vi "Main.vi"() -> ()   [LabVIEW 2020]
uses:
  System.Windows.Forms
  Global_Variable/Global.vi
  Global_Variable/A131258.vi
  Database/Global1.vi
  <userlib>/_MGI/Menu Building/MenuTypes/MenuStrip/MGI_MenuStrip.lvclass
  <userlib>/_MGI/Menu Building/MenuItemStatusChange/MGI_MenuItemStatusChange.lvclass
  Libraries/S7/S7.lvlib
panel:
  out "左空载扭矩":dbl format="%#.3f Nm"
  out "右加载扭矩":dbl format="%#.3f Nm"
  out "上序状态":string
  out "右工位传感器码":string
  in  "表格控件":string[][](table)
  in  "Andon":enum32{"未选择", "缺料报警", "质量报警", "故障报警"}(radio)
  out "PLC":bool
  in  "菜单":refnum<k24>(container)
  out "试验计时":u16
  out "工位传感器码":string
  out "生产数量":i32
  out "合格数量":i32
  out "userStatus":string caption="用户状态"
  out "userName":string caption="用户名"
  out "connectionMode":string caption="联机类型"
  out "产品型号":string
  in  "更换产品":refnum<vi>
  out "提示信息":string
  out "错误":bool
  out "时间字符串":string
  out "日期字符串":string
  out "自动":bool
  # "芯轴分总成磨合台"
  # "实验项目"
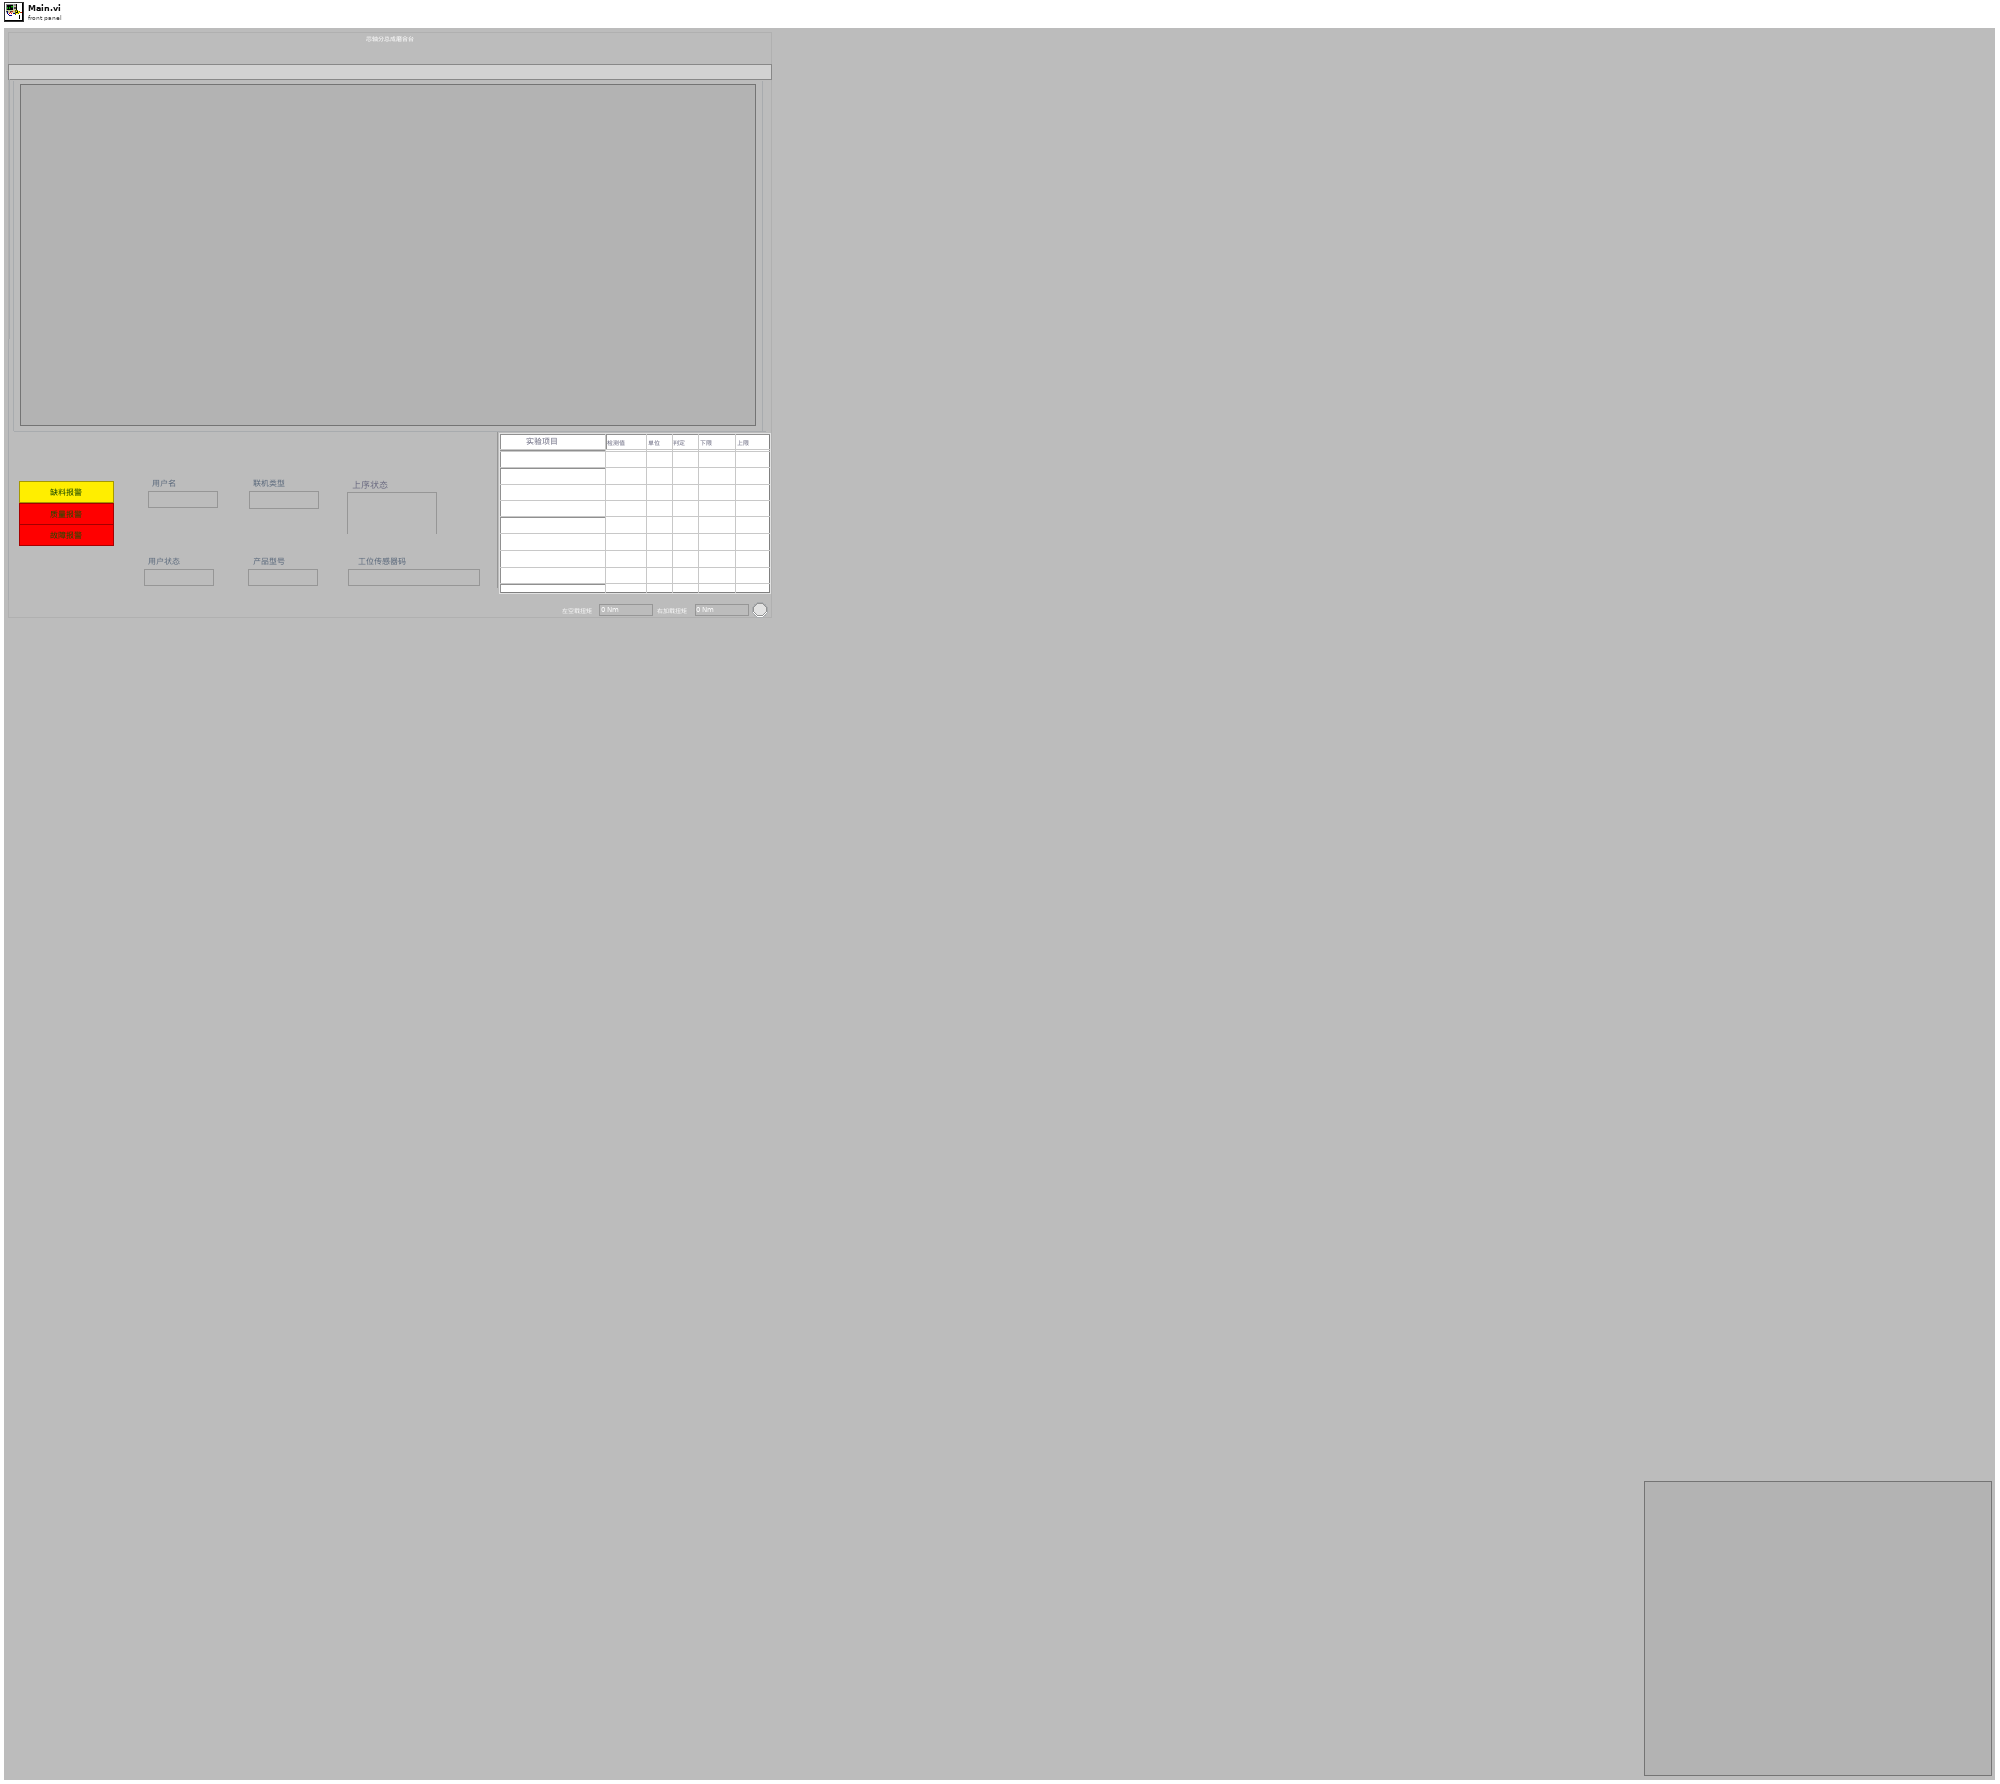
[diagram p1: front panel]
types:
  T1 = typedef "S7.lvlib/Broadcast Events--cluster.ctl" = cluster{"Module Did Init":refnum<user-event>, "Status Updated":refnum<user-event>, "Error Reported":refnum<user-event>, "Module Did Stop":refnum<user-event>, "Update Module Execution Status":refnum<user-event>}
  T2 = enum32{"Invalid", "Standard", "Closed", "Hidden", "Minimized", "Maximized"}
  T3 = cluster{"设备名称":string, "操作人员":string, "设备状态":enum16{"设备离线", "设备正常", "设备缺料", "设备故障", "质量报警"}, "附加信息":string}
  T4 = enum32{"invalid app kind", "Development System", "Run Time System", "Student Edition", "Embedded LabVIEW", "Evaluation", "Custom"}
  T5 = cluster{"左平均扭矩":cluster{"正转":dbl, "反转":dbl}, "左矩波动":cluster{"正转":dbl, "反转":dbl}, "左空载":cluster{"正转":dbl, "反转":dbl}, "右平均扭矩":cluster{"正转":dbl, "反转":dbl}, "右扭矩波动":cluster{"正转":dbl, "反转":dbl}, "右空载":cluster{"正转":dbl, "反转":dbl}, "扭矩对称":cluster{"左":dbl, "右":dbl}, "左零点漂移":cluster{"正":dbl, "反":dbl}, "右零点漂移":cluster{"正":dbl, "反":dbl}}
  T6 = cluster{"用户编号":string, "用户名":string, "用户密码(密文)":string, "用户权限":string}
  T7 = cluster{"Core":cluster{"Current VI Reference":refnum<vi>, "Close Panel on Exit?":bool}, "Your Boolean data":bool, "Your string data":string}
  T8 = cluster{"Current VI Reference":refnum<vi>, "Close Panel on Exit?":bool}
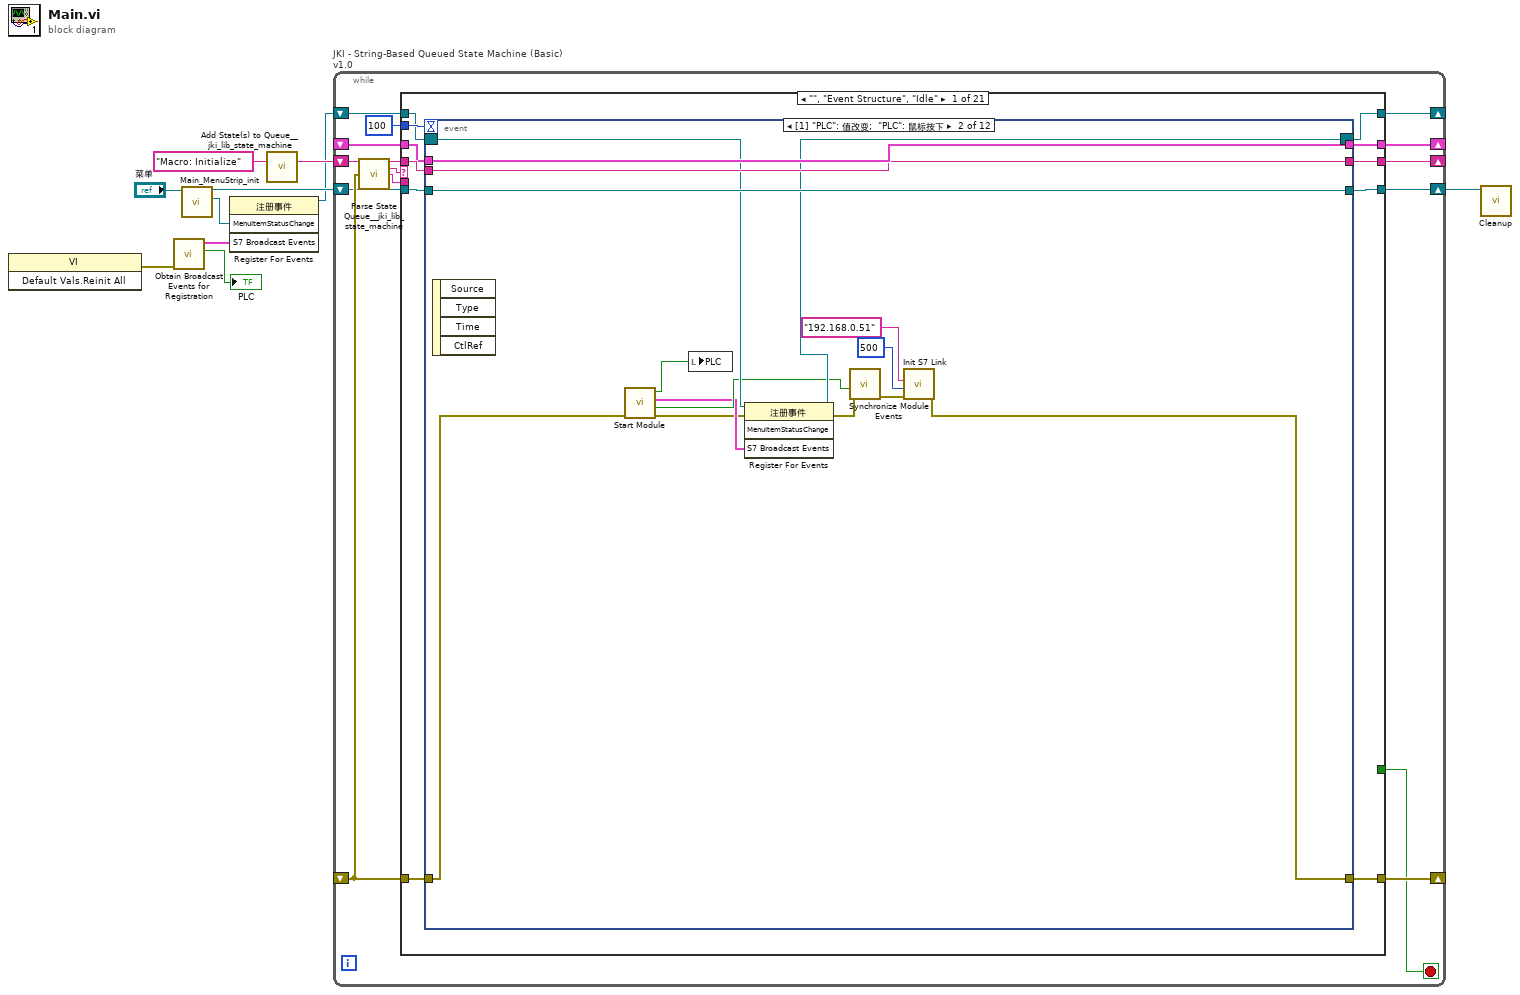
[diagram p0: block diagram]
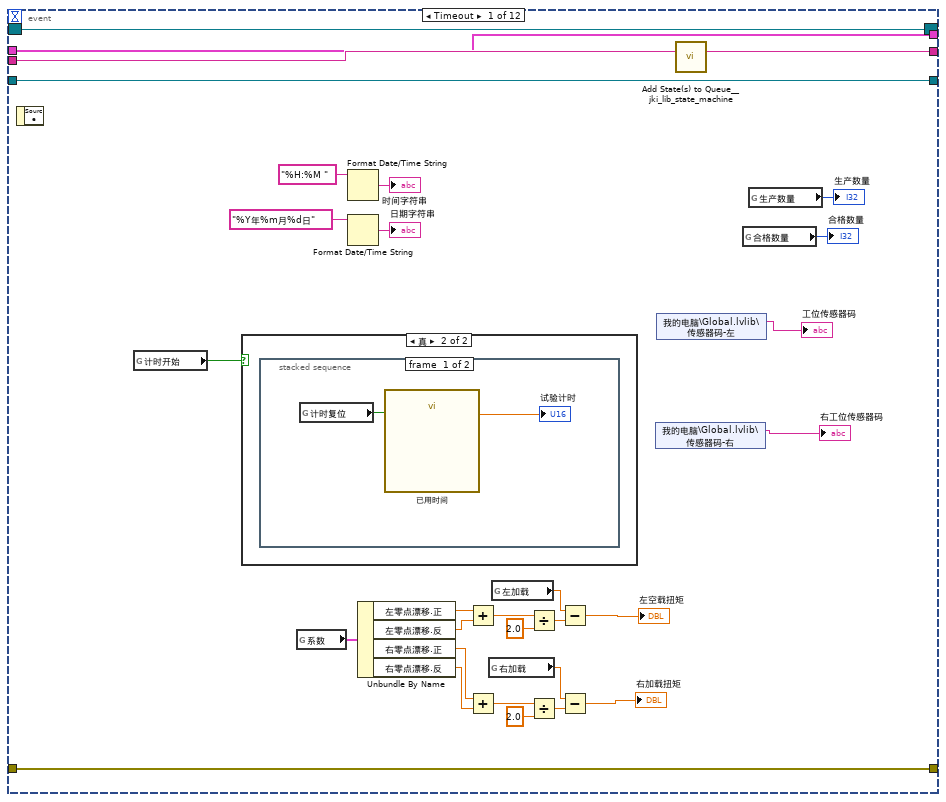
[diagram p2: hidden frame]
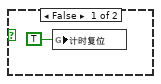
[diagram p3: hidden frame]
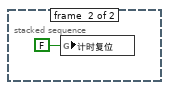
[diagram p4: hidden frame]
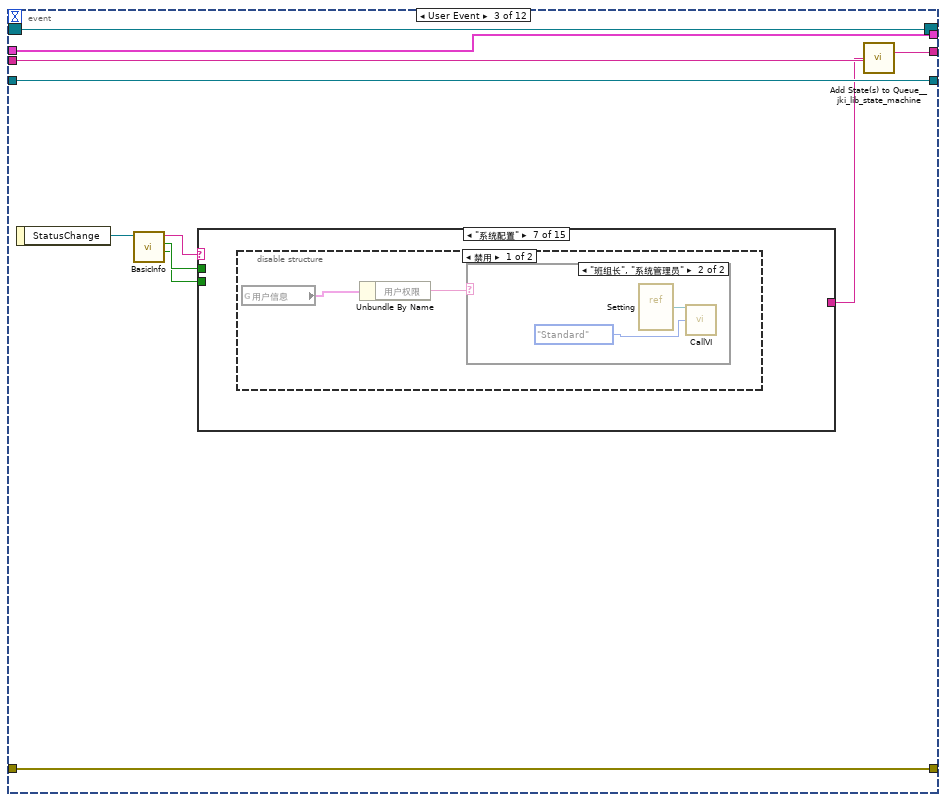
[diagram p5: hidden frame]
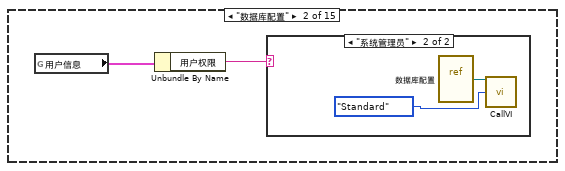
[diagram p7: hidden frame]
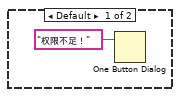
[diagram p8: hidden frame]
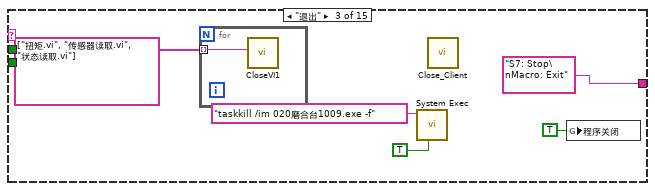
[diagram p9: hidden frame]
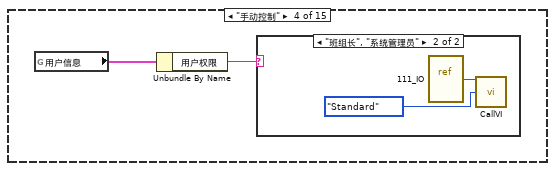
[diagram p10: hidden frame]
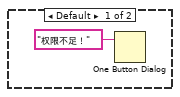
[diagram p11: hidden frame]
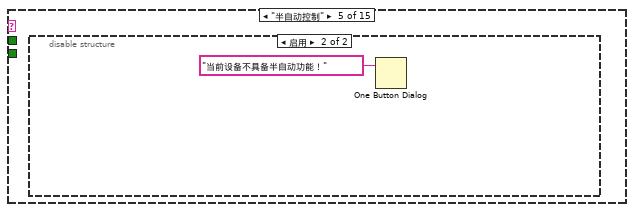
[diagram p12: hidden frame]
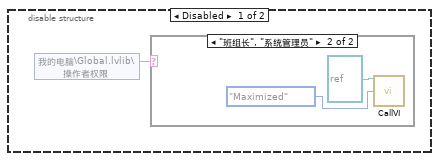
[diagram p13: hidden frame]
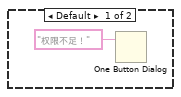
[diagram p14: hidden frame]
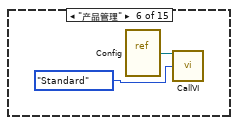
[diagram p15: hidden frame]
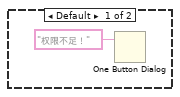
[diagram p16: hidden frame]
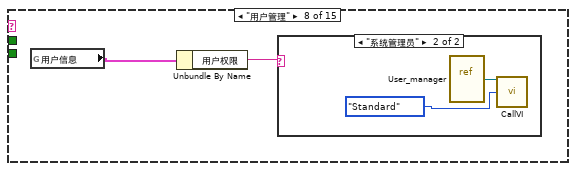
[diagram p18: hidden frame]
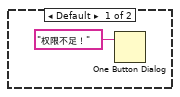
[diagram p19: hidden frame]
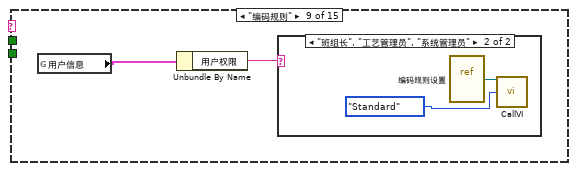
[diagram p20: hidden frame]
diagram:
  n1 = invoke class="VI" method="Default Vals.Reinit All"() -> (error out=w3:errorcluster)  [unwired: 3 in, 2 out]
  n2 = call "Obtain Broadcast Events for Registration.vi"("error in (no error)"=w3) -> ("Already running?"=→"PLC":bool, "S7 Broadcast Events"=w5:T1)  [unwired: 8 in, 1 out]
  n3 = call "Main_MenuStrip_init.vi"("MenuStrip"="菜单") -> ("MenuItemStatusChange"=w2:refnum<user-event>, "Menu out"=w7:refnum<class "MGI_MenuStrip.lvclass">)  [unwired: 9 in]
  n4 = register-events(w2, w5) -> (reference out=w1:refnum<event-registration>)  [unwired: 2 in, 1 out]
  n5 = call <vilib>:"Add State(s) to Queue__jki_lib_state_machine.vi"("State(s) in (\"\")"="Macro: Initialize") -> ("States Out"=w10:string)  [unwired: 14 in]
  n6 = while "JKI - String-Based Queued State Machine (Basic) v1.0" {
    shift-right: [w19] -> _
    shift-left: _ -> [w18]
    shift-right: [w21] -> _
    shift-left: _ -> [w16]
    shift-right: [w20] -> _
    shift-left: w10 -> [w22]
    shift-right: [w14] -> w6
    shift-left: w7 -> [w15]
    shift-right: [w12] -> _
    shift-left: w1 -> [w11]
    stop <- w13 stop-if-true
    n7 = call <vilib>:"Parse State Queue__jki_lib_state_machine.vi"("State Queue"=w22, "Error In (no error)"=w16) -> ("Remaining States"=w24:string, "Current State"=w25:string, "Arguments"=w23:string)  [unwired: 11 in]
    n8 = case shown="\"\", \"Event Structure\", \"Idle\"" w25 {
      selector: w25 -> [_ _ w254 _ _ _ _ _ _ _ _ _ _ _ _ _ _ _ _ _ _]
      tunnel: w24 -> [w36 w251 w258 w278 w286 w293 w299 w303 w309 w318 w329 w337 w343 w356 w380 w416 w424 w437 w465 w472 w484]
      tunnel: w23 -> [_ _ _ _ _ _ _ _ _ _ _ _ _ _ _ _ w419 w431 _ _ _]
      tunnel: w18 -> [w34 w248 w256 w269 w283 w291 w296 w304 w312 w315 _ w332 w340 w354 w378 w413 w422 w433 w462 w469 w481]
      tunnel: [w33 w249 w260 w275 errorcluster {"status"=FALSE, "code"=0, "source"=""} ("error out") w290 w297 w301 w307 w316 w326 w333 w341 w353 w376 w414 w420 w434 w463 w470 w482] -> w21
      tunnel: w16 -> [w32 w249 w259 w275 w282 w290 w297 w301 w308 w316 w326 w334 w341 w350 w376 w414 w421 w435 w463 w470 w482]
      tunnel: [w35 w250 w257 w277 w285 w292 w298 w303 w310 w317 w328 w336 w342 w355 w379 w415 w423 w436 w464 w471 w483] -> w20
      tunnel: [w31 w248 w256 w276 w283 w291 w296 w304 w312 w315 w327 w332 w340 w354 w378 w413 w422 w433 w462 w469 w481] -> w19
      tunnel: 100 ("Timeout") -> [w30 _ _ _ _ _ _ _ _ _ _ _ _ _ _ _ _ _ _ _ _]
      tunnel: w15 -> [w29 w247 w253 w266 w280 w289 w295 w302 w311 w314 w321 w331 w339 w352 w377 w412 w418 w430 w461 w467 w474]
      tunnel: [w28 w247 w253 w266 w280 w289 w295 w302 w311 w314 w321 w331 w339 w352 w377 w412 w418 w430 w461 w467 w474] -> w14
      tunnel: [_ _ _ _ _ TRUE _ _ _ _ _ _ _ _ _ _ _ _ _ _ _] -> w13
      tunnel: [w26 w246 w252 w265 w279 w287 w294 w305 w306 w313 w322 w330 w338 w351 w375 w409 w417 w429 w460 w466 w473] -> w12
      tunnel: w11 -> [w27 w246 w252 w265 w279 w287 w294 w305 w306 w313 w322 w330 w338 w351 w375 w409 w417 w429 w460 w466 w473]
      frame "", "Event Structure", "Idle" {
        n9 = event shown="[1] \"PLC\": 值改变;  \"PLC\": 鼠标按下" {
          selector: w27 -> [w56 w80 w86 w156 w163 w170 w177 w191 w200 w208 w216 _]
          dyn-events: [w56 w79 w86 w156 w163 w170 w177 w191 w200 w208 w216 _] -> w26
          timeout: w30 -> [_ _ _ _ _ _ _ _ _ _ _ _]
          tunnel: w36 -> [w66 w84 w95 w157 w164 w173 w180 w188 w204 w214 w218 w240]
          tunnel: [w65 w84 w93 w158 w165 w174 w181 w189 w205 w213 w219 w240] -> w35
          tunnel: w34 -> [w64 w85 w94 w160 w168 w175 w182 w190 w206 w211 w221 w241]
          tunnel: [w57 w81 w96 w161 w166 w171 w183 w186 w203 w212 w220 w238] -> w33
          tunnel: w32 -> [w57 w82 w96 w161 w166 w171 w184 w186 w203 w212 w220 w238]
          tunnel: [w64 w85 w94 w160 w168 w175 w182 w190 w206 w211 w221 w241] -> w31
          tunnel: w29 -> [w55 w83 w89 w159 w167 w172 w179 w187 _ _ _ w239]
          tunnel: [w55 w83 w89 w159 w167 w172 w179 w187 _ _ _ w239] -> w28
          event Timeout {
            n10 = event-data() -> ()  [unwired: 1 in, 1 out]
            n11 = global read "Global.vi" "计时开始"() -> (w54:bool)
            n12 = case shown="真" w54 {
              frame False {
                n13 = global write "Global.vi" "计时复位"(TRUE ("计时复位")) -> ()
              }
              frame True {
                n14 = stacked-sequence {
                  frame #0 {
                    n15 = global read "Global.vi" "计时复位"() -> (w68:bool)
                    n16 = call "已用时间"("Reset"=w68) -> ("Elapsed Time (s)"=→"试验计时":dbl)  [unwired: 11 in, 7 out]
                  }
                  frame #1 {
                    n17 = global write "Global.vi" "计时复位"(FALSE ("计时复位")) -> ()
                  }
                }
              }
            }
            n18 = global read "A131258.vi" "系数"() -> (w51:T5)
            n19 = Format Date/Time String(time format string (%c)="%H:%M ") -> (date/time string=→"时间字符串":string)  [unwired: 2 in]
            n20 = Format Date/Time String(time format string (%c)="%Y年%m月%d日") -> (date/time string=→"日期字符串":string)  [unwired: 2 in]
            n21 = Unbundle By Name(w51) -> ("左零点漂移.正"=w50:dbl, "左零点漂移.反"=w49:dbl, "右零点漂移.正"=w42:dbl, "右零点漂移.反"=w41:dbl)
            n22 = Add(x=w50, y=w49) -> (x+y=w48:dbl)
            n23 = Add(x=w42, y=w41) -> (x+y=w43:dbl)
            n24 = global read "全局2.vi" "右加载"() -> (w40:dbl)
            n25 = global read "全局1.vi" "左加载"() -> (w46:dbl)
            n26 = Divide(x=w48, y=2.0) -> (x/y=w47:dbl)
            n27 = Divide(x=w43, y=2.0) -> (x/y=w44:dbl)
            n28 = Subtract(x=w46, y=w47) -> (x-y=→"左空载扭矩":dbl)
            n29 = Subtract(x=w40, y=w44) -> (x-y=→"右加载扭矩":dbl)
            n30 = shared-variable "我的电脑\\Global.lvlib\\传感器码-右"() -> (→"右工位传感器码":string)  [unwired: 1 in, 1 out]
            n31 = shared-variable "我的电脑\\Global.lvlib\\传感器码-左"() -> (→"工位传感器码":string)  [unwired: 1 in, 1 out]
            n32 = call <vilib>:"Add State(s) to Queue__jki_lib_state_machine.vi"("State(s) in (\"\")"=w66) -> ("States Out"=w65:string)  [unwired: 14 in]
            n33 = global read "Global.vi" "合格数量"() -> (→"合格数量":i32)
            n34 = global read "Global.vi" "生产数量"() -> (→"生产数量":i32)
          }
          event "PLC": Value Change; "PLC": Mouse Down {
            n35 = event-data() -> ()  [unwired: 1 in, 4 out]
            n36 = call "Start Module.vi"("error in (no error)"=w82) -> ("error out"=w75:errorcluster, "Wait for Event Sync?"=w78:bool, "S7 Broadcast Events"=w77:T1, "Module Was Already Running?"=w76:bool)  [unwired: 7 in]
            n37 = local write "PLC"(w76) -> ()
            n38 = register-events(reference=w80, error in=w75, w77) -> (reference out=w79:refnum<event-registration>, error out=w74:errorcluster)  [unwired: 1 in]
            n39 = call "Synchronize Module Events.vi"("error in (no error)"=w74, "Wait for Event Sync?"=w78) -> ("error out"=w71:errorcluster)  [unwired: 9 in]
            n40 = call "Init S7 Link.vi"("error in (no error)"=w71, "超时"=500, "IP"="192.168.0.51") -> ("error out"=w81:errorcluster)  [unwired: 8 in]
          }
          event User Event {
            n41 = event-data() -> ("StatusChange"=w87:refnum<class "MGI_MenuItemStatusChange.lvclass">)  [unwired: 1 in]
            n42 = call <userlib>:"BasicInfo.vi"("MGI_MenuItemStatusChange in"=w87) -> ("Enabled?"=w90:bool, "Checked?"=w91:bool, "Tag"=w92:string)  [unwired: 7 in, 1 out]
            n43 = case shown="\"系统配置\"" w92 {
              tunnel: w91 -> [_ _ _ _ _ _ _ _ _ _ _ _ _ _ _]
              tunnel: w90 -> [_ _ _ _ _ _ _ _ _ _ _ _ _ _ _]
              tunnel: [_ _ "S7: Stop\nMacro: Exit" _ _ _ _ _ _ _ _ _ _ _ _] -> w88
              frame "假", Default {
              }
              frame "数据库配置" {
                n44 = global read "Global1.vi" "用户信息"() -> (w97:T6)
                n45 = Unbundle By Name(w97) -> ("用户权限"=w98:string)
                n46 = case shown="\"系统管理员\"" w98 {
                  frame Default {
                    n47 = One Button Dialog(message="权限不足！" ("消息")) -> ()  [unwired: 1 in, 1 out]
                  }
                  frame "系统管理员" {
                    n48 = vi-ref "数据库配置.vi"() -> (w101:refnum<vi>)
                    n49 = call "CallVI.vi"("VI引用"=w101, "状态"=T2."Standard") -> ()  [unwired: 11 in, 3 out]
                  }
                }
              }
              frame "退出" {
                n50 = for {
                  tunnel: string[] ["扭矩.vi", "传感器读取.vi", "状态读取.vi"] -> [w107] mode=indexing
                  n51 = call "CloseVI1.vi"("名称或相对路径"=w107) -> ()  [unwired: 10 in, 1 out]
                }
                n52 = call <vilib>:"System Exec.vi"("run minimized? (F)"=TRUE, "command line"="taskkill /im 020磨合台1009.exe -f") -> ()  [unwired: 6 in, 4 out]
                n53 = call "Close_Client.vi"() -> ()  [unwired: 12 in]
                n54 = global write "Global.vi" "程序关闭"(TRUE ("程序关闭")) -> ()
              }
              frame "手动控制" {
                n55 = global read "Global1.vi" "用户信息"() -> (w108:T6)
                n56 = Unbundle By Name(w108) -> ("用户权限"=w109:string)
                n57 = case shown="\"班组长\", \"系统管理员\"" w109 {
                  frame Default {
                    n58 = One Button Dialog(message="权限不足！" ("消息")) -> ()  [unwired: 1 in, 1 out]
                  }
                  frame "班组长", "系统管理员" {
                    n59 = vi-ref "111_IO.vi"() -> (w112:refnum<vi>)
                    n60 = call "CallVI.vi"("VI引用"=w112, "状态"=T2."Standard") -> ()  [unwired: 11 in, 3 out]
                  }
                }
              }
              frame "半自动控制" {
                n61 = disable-structure shown="启用" {
                  frame Disabled {
                    n62 = shared-variable "我的电脑\\Global.lvlib\\操作者权限"() -> (w113:string)  [unwired: 1 in, 1 out]
                    n63 = case shown="\"班组长\", \"系统管理员\"" w113 {
                      frame Default {
                        n64 = One Button Dialog(message="权限不足！" ("消息")) -> ()  [unwired: 1 in, 1 out]
                      }
                      frame "班组长", "系统管理员" {
                        n65 = call "CallVI.vi"("VI引用"=refnum<vi> refnum, "状态"=T2."Maximized") -> ()  [unwired: 11 in, 3 out]
                      }
                    }
                  }
                  frame Enabled {
                    n66 = One Button Dialog(message="当前设备不具备半自动功能！" ("消息")) -> ()  [unwired: 1 in, 1 out]
                  }
                }
              }
              frame "产品管理" {
                n67 = vi-ref "Config.vi"() -> (w119:refnum<vi>)
                n68 = call "CallVI.vi"("VI引用"=w119, "状态"=T2."Standard") -> ()  [unwired: 11 in, 3 out]
              }
              frame "系统配置" {
                n69 = disable-structure shown="禁用" {
                  frame Disabled {
                    n70 = global read "Global1.vi" "用户信息"() -> (w120:T6)
                    n71 = Unbundle By Name(w120) -> ("用户权限"=w121:string)
                    n72 = case shown="\"班组长\", \"系统管理员\"" w121 {
                      frame Default {
                        n73 = One Button Dialog(message="权限不足！" ("消息")) -> ()  [unwired: 1 in, 1 out]
                      }
                      frame "班组长", "系统管理员" {
                        n74 = vi-ref "Setting.vi"() -> (w124:refnum<vi>)
                        n75 = call "CallVI.vi"("VI引用"=w124, "状态"=T2."Standard") -> ()  [unwired: 11 in, 3 out]
                      }
                    }
                  }
                  frame Enabled {
                  }
                }
              }
              frame "用户管理" {
                n76 = global read "Global1.vi" "用户信息"() -> (w125:T6)
                n77 = Unbundle By Name(w125) -> ("用户权限"=w126:string)
                n78 = case shown="\"系统管理员\"" w126 {
                  frame Default {
                    n79 = One Button Dialog(message="权限不足！" ("消息")) -> ()  [unwired: 1 in, 1 out]
                  }
                  frame "系统管理员" {
                    n80 = vi-ref "User_manager.vi"() -> (w129:refnum<vi>)
                    n81 = call "CallVI.vi"("VI引用"=w129, "状态"=T2."Standard") -> ()  [unwired: 11 in, 3 out]
                  }
                }
              }
              frame "编码规则" {
                n82 = global read "Global1.vi" "用户信息"() -> (w130:T6)
                n83 = Unbundle By Name(w130) -> ("用户权限"=w131:string)
                n84 = case shown="\"班组长\", \"工艺管理员\", \"系统管理员\"" w131 {
                  frame Default {
                    n85 = One Button Dialog(message="权限不足！" ("消息")) -> ()  [unwired: 1 in, 1 out]
                  }
                  frame "班组长", "工艺管理员", "系统管理员" {
                    n86 = vi-ref "编码规则设置.vi"() -> (w134:refnum<vi>)
                    n87 = call "CallVI.vi"("VI引用"=w134, "状态"=T2."Standard") -> ()  [unwired: 11 in, 3 out]
                  }
                }
              }
              frame "易损件管理" {
                n88 = vi-ref "易损件管理.vi"() -> (w136:refnum<vi>)
                n89 = call "CallVI.vi"("VI引用"=w136, "状态"=T2."Standard") -> ()  [unwired: 11 in, 3 out]
              }
              frame "物料批次管理" {
                n90 = vi-ref "批次管理.vi"() -> (w138:refnum<vi>)
                n91 = call "CallVI.vi"("VI引用"=w138, "状态"=T2."Standard") -> ()  [unwired: 11 in, 3 out]
              }
              frame "报表" {
                n92 = call "文件对话框"("start path"=path "D:/report", "prompt"="打开报表", "pattern (all files)"="*.doc;*.docx", "pattern label"="Word 文档") -> ("selected path"=w139:path, "error out"=w140:errorcluster)  [unwired: 8 in, 2 out]
                n93 = case shown="无错误" w140 {
                  selector: w140 -> [w146 w148]
                  tunnel: w139 -> [w147 _]
                  frame No Error {
                    w145 = 1 items=["Normal", "Maximize", "Minimize"] ("cpubbs_WindowState")
                    n94 = call "Open_Word.vi"("File Path"=w147, "cpubbs_WindowState"=w145, "错误输入（无错误）"=w146) -> ()  [unwired: 12 in, 1 out]
                  }
                  frame Error {
                    n95 = call <vilib>:"Clear Errors.vi"("error in (no error)"=w148) -> ()  [unwired: 5 in, 2 out]
                  }
                }
              }
              frame "报警信息" {
                n96 = vi-ref "报警信息.vi"() -> (w150:refnum<vi>)
                n97 = call "CallVI.vi"("VI引用"=w150, "状态"=T2."Standard") -> ()  [unwired: 11 in, 3 out]
              }
              frame "关于" {
                n98 = vi-ref "About.vi"() -> (w152:refnum<vi>)
                n99 = call "CallVI.vi"("VI引用"=w152, "状态"=T2."Standard") -> ()  [unwired: 11 in, 3 out]
              }
              frame "操作演示" {
                n100 = call <vilib>:"Application Directory.vi"() -> ("Application Directory"=w155:path)
                n101 = Build Path(base path=w155, name or relative path="操作演示" ("名称或相对路径")) -> (appended path=w154:path)
                n102 = call "自动播放ppt.vi"("路径"=w154) -> ()  [unwired: 10 in, 1 out]
              }
            }
            n103 = call <vilib>:"Add State(s) to Queue__jki_lib_state_machine.vi"("State(s) in (\"\")"=w95, "State(s) at Back (\"\")"=w88) -> ("States Out"=w93:string)  [unwired: 13 in]
          }
          event User Event {
            n104 = event-data() -> ("Init?"=w162:bool)  [unwired: 1 in, 1 out]
            n105 = local write "PLC"(w162) -> ()
            n106 = call <vilib>:"Add State(s) to Queue__jki_lib_state_machine.vi"("State(s) in (\"\")"=w157) -> ("States Out"=w158:string)  [unwired: 14 in]
          }
          event User Event {
            n107 = event-data() -> ("Running?"=w169:bool)  [unwired: 1 in]
            n108 = local write "PLC"(w169) -> ()
            n109 = call <vilib>:"Add State(s) to Queue__jki_lib_state_machine.vi"("State(s) in (\"\")"=w164) -> ("States Out"=w165:string)  [unwired: 14 in]
          }
          event User Event {
            n110 = event-data() -> ()  [unwired: 1 in, 7 out]
            n111 = local write "PLC"(FALSE ("PLC")) -> ()
            n112 = call <vilib>:"Add State(s) to Queue__jki_lib_state_machine.vi"("State(s) in (\"\")"=w173) -> ("States Out"=w174:string)  [unwired: 14 in]
          }
          event User Event {
            n113 = event-data() -> ("Error"=w185:errorcluster)  [unwired: 1 in]
            n114 = Merge Errors(w185, w184) -> (w183:errorcluster)
            n115 = call <vilib>:"Add State(s) to Queue__jki_lib_state_machine.vi"("State(s) in Front (\"\")"="S7: Initialize\nIdle", "State(s) in (\"\")"=w180) -> ("States Out"=w181:string)  [unwired: 13 in]
          }
          event "自动": Mouse Down {
            n116 = event-data() -> ()  [unwired: 1 in, 1 out]
            n117 = disable-structure shown="禁用" {
              frame Disabled {
                n118 = local read "自动"() -> (w192:bool)
                n119 = case shown="假" w192 {
                  frame False {
                    n120 = call "设备状态.vi"() -> ("Status_Read"=w193:i16)  [unwired: 11 in]
                    n121 = case shown="5" w193 {
                      frame 0, Default {
                        n122 = One Button Dialog(message="请复位！" ("消息")) -> ()  [unwired: 1 in, 1 out]
                      }
                      frame 5 {
                      }
                    }
                  }
                  frame True {
                    n123 = Two Button Dialog(message="确定要退出自动？" ("消息")) -> (T button?=w195:bool)  [unwired: 2 in]
                    n124 = case shown="真" w195 {
                      frame False {
                      }
                      frame True {
                        n125 = vi-ref "Auto.vi"() -> (w199:refnum<vi>)
                        n126 = invoke class="VI" method="Ctrl Val.Set"(reference=w199, "Control Name"="STEP" ("控件名"), "Value"="退出自动" ("控件名")) -> ()  [unwired: 2 in, 5 out]
                      }
                    }
                  }
                }
              }
              frame Enabled {
              }
            }
            n127 = call <vilib>:"Add State(s) to Queue__jki_lib_state_machine.vi"("State(s) in (\"\")"=w188) -> ("States Out"=w189:string)  [unwired: 14 in]
          }
          event "错误": Mouse Down {
            n128 = event-data() -> ()  [unwired: 1 in, 8 out]
            n129 = vi-ref "报警信息.vi"() -> (w202:refnum<vi>)
            n130 = call "CallVI.vi"("VI引用"=w202, "状态"=T2."Standard") -> ()  [unwired: 11 in, 3 out]
            n131 = call <vilib>:"Add State(s) to Queue__jki_lib_state_machine.vi"("State(s) in (\"\")"=w204) -> ("States Out"=w205:string)  [unwired: 14 in]
          }
          event Panel Close? {
            w207 = TRUE ("程序关闭")
            n132 = event-data() -> ()  [unwired: 1 in, 1 out]
            n133 = global write "Global.vi" "程序关闭"(w207) -> ()
            n134 = call <vilib>:"Add State(s) to Queue__jki_lib_state_machine.vi"("State(s) in Front (\"\")"="S7: Stop\nMacro: Exit", "State(s) in (\"\")"=w214) -> ("States Out"=w213:string)  [unwired: 13 in]
            n135 = Quit LabVIEW(quit? (T)=w207) -> ()
            n136 = event-data("Discard?"=TRUE) -> ()  [unwired: 1 in, 1 out]
          }
          event "更换产品": Value Change {
            n137 = event-data() -> ("NewVal"=w217:refnum<vi>)  [unwired: 1 in, 5 out]
            n138 = stacked-sequence {
              tunnel: w217 -> [w230]
              tunnel: ["Idle"] -> w215
              frame #0 {
                n139 = disable-structure shown="禁用" {
                  disable-tunnel: w230 -> [w232 _]
                  frame Disabled {
                    n140 = control-ref of="子面板"() -> (w231:refnum<vi>)
                    n141 = call "Call_SubPanal.vi"("VI引用句柄"=w232, "SubPnl引用句柄"=w231) -> ()  [unwired: 9 in, 1 out]
                  }
                  frame Enabled {
                  }
                }
                n142 = vi-ref "Auto.vi"() -> (w227:refnum<vi>)
                n143 = invoke class="VI" method="Ctrl Val.Get"(reference=w227, "Control Name"="标尺_Event" ("控件名")) -> ("Get Control Value Variant"=w226:variant)  [unwired: 2 in, 3 out]
                n144 = shared-variable "我的电脑\\Global.lvlib\\产品型号"() -> (w222:string)  [unwired: 1 in, 1 out]
                n145 = Variant To Data(type=refnum<user-event> refnum ("标尺_Event"), Variant=w226) -> (data=w223:refnum<user-event>, error out=w224:errorcluster)  [unwired: 1 in]
                n146 = Generate User Event(user event=w223, event data cluster=w222, error in=w224) -> ()  [unwired: 1 in, 2 out]
                n147 = local write "产品型号"(w222) -> ()
              }
            }
            n148 = call <vilib>:"Add State(s) to Queue__jki_lib_state_machine.vi"("State(s) in Front (\"\")"=w215, "State(s) in (\"\")"=w218) -> ("States Out"=w219:string)  [unwired: 13 in]
          }
          event "Andon": Value Change {
            n149 = event-data() -> ("NewVal"=w237:enum32{"未选择", "缺料报警", "质量报警", "故障报警"})  [unwired: 1 in]
            n150 = case shown="\"故障报警\"" w237 {
              tunnel: [enum16{"设备离线", "设备正常", "设备缺料", "设备故障", "质量报警"}."设备正常" ("设备状态") enum16{"设备离线", "设备正常", "设备缺料", "设备故障", "质量报警"}."设备缺料" ("设备状态") enum16{"设备离线", "设备正常", "设备缺料", "设备故障", "质量报警"}."质量报警" ("设备状态") enum16{"设备离线", "设备正常", "设备缺料", "设备故障", "质量报警"}."设备故障" ("设备状态")] -> w235
              frame "未选择", Default {
              }
              frame "缺料报警" {
              }
              frame "质量报警" {
              }
              frame "故障报警" {
              }
            }
            n151 = local read "userName"() -> (w234:string)
            n152 = Bundle By Name(cluster=T3 {"设备名称"="芯轴分总成磨合台", "操作人员"="", "设备状态"=enum."设备离线", "附加信息"=""} ("设备信息"), "操作人员"=w234, "设备状态"=w235) -> (w233:T3)
            n153 = call "Change_Client.vi"("设备信息"=w233) -> ()  [unwired: 10 in, 1 out]
          }
        }
      }
      frame "---------- Core ----------" {
        n154 = call <vilib>:"Add State(s) to Queue__jki_lib_state_machine.vi"("State(s) in (\"\")"=w251) -> ("States Out"=w250:string)  [unwired: 14 in]
      }
      frame Default {
        w263 = 42 items=["No error", "Argument error", "Memory is full", "Out of zone", "End of file", "File already open", "Generic file I/O error", "File not found", "File permission error", "Disk is full", "Duplicate path", "Too many files open", "System feature not enabled", "Resource file not found", "Cannot add resource", "Resource not found", "Image not found", "Image memory error", "Pen does not exist", "Config type invalid", "Config token not found", "Config parse error", "Config memory error", "Bad external code format", "Bad external code offset", "External code not present", "Null window", "Destroy window error", "Null menu", "Print aborted", "Bad print record", "Print driver error", "Windows error during printing", "Memory error during printing", "Print dialog error", "Generic print error", "Invalid device refnum", "Device not found", "Device parameter error", "Device unit error", "Cannot open device", "Device call aborted", "Generic error", "Cancelled by user", "Object ID too low", "Object ID too high", "Object not in heap", "Unknown heap", "Unknown object (invalid DefProc)", "Unknown object (DefProc not in table)", "Message out of range", "Invalid (null) method", "Unknown message", "Manager call not supported", "Bad address", "Network operation in progress", "Network operation timed out", "Connection is busy", "Network attribute not supported", "Network error", "Address in use", "System out of memory", "Connection aborted", "Connection refused", "Not connected", "Already connected", "Connection closed", "Initialization error (interapplication manager)", "Bad occurrence", "Wait on unbound occurrence handler", "Occurrence queue overflow", "Datalog type conflict", "Unused", "Unrecognized type (interapplication manager)", "Memory corrupt", "Failed to make temporary DLL", "Old CIN version", "Drag socket not found", "Failed to load drop-object", "Failed to register OLE object", "Failed to release OLE object", "Format specifier type mismatch", "Unknown format specifier", "Too few format specifiers", "Too many format specifiers", "Scan failed", "Newer CIN version", "Error converting to variant", "Runtime menu error", "Password tampered", "Variant attribute not found", "Incompatible variant data type", "Event data is not available", "Event Store is not present", "Occurrence is not found", "Event Queue is not created", "Event info is not available", "Refnum passed is NULL", "Error retrieving Class GUID", "Error retrieving CoClass GUID", "Error retrieving TypeLib GUID.", "Bad built application magic bytes.", "Specific driver is different from the specific driver associated with the Logical Name.", "There is no session opened to the class driver.", "Max Error", "MAX - Error with config objects", "MAX - Error loading configuration", "MAX - Group not supported"]
        # "Current State"
        n155 = Format Into String(format string="Software Exception: Unhandled State \"%s\"." ("message"), error in=w259, w254) -> (resulting string=w262:string, error out=w261:errorcluster)  [unwired: 1 in]
        n156 = call <vilib>:"Error Cluster From Error Code.vi"("show call chain? (False)"=TRUE, "error in (no error)"=w261, "error message (\"\")"=w262, "error code (0)"=w263) -> ("error out"=w260:errorcluster)  [unwired: 5 in]
        n157 = call <vilib>:"Add State(s) to Queue__jki_lib_state_machine.vi"("State(s) in (\"\")"=w258) -> ("States Out"=w257:string)  [unwired: 14 in]
      }
      frame "Initialize Core Data" {
        # "originally closed?"
        # "exe?"
        n158 = property class="VI"() -> ("Front Panel.Open"=w274:bool)  [unwired: 2 in, 2 out]
        n159 = property class="App"() -> ("App.Kind"=w273:T4)  [unwired: 2 in, 2 out]
        n160 = control-ref of="Current VI Reference"() -> (w267:refnum<vi>)
        n161 = Not(x=w274) -> (.not. x?=w271:bool)
        n162 = Equal?(x=w273, y=T4."Run Time System" ("Application:Kind")) -> (x = y?=w270:bool)
        n163 = Or(x=w271, y=w270) -> (x .or. y?=w268:bool)
        n164 = Bundle By Name(cluster=w269, "Core.Current VI Reference"=w267, "Core.Close Panel on Exit?"=w268) -> (w276:T7)
        n165 = call <vilib>:"Add State(s) to Queue__jki_lib_state_machine.vi"("State(s) in (\"\")"=w278) -> ("States Out"=w277:string)  [unwired: 14 in]
      }
      frame "Error Handler" {
        n166 = call <vilib>:"General Error Handler.vi"("error in (no error)"=w282) -> ()  [unwired: 10 in, 5 out]
        n167 = call <vilib>:"Add State(s) to Queue__jki_lib_state_machine.vi"("State(s) in Front (\"\")"="/* Post Error States", "State(s) in (\"\")"=w286) -> ("States Out"=w285:string)  [unwired: 13 in]
      }
      frame "Exit" {
        n168 = call <vilib>:"Add State(s) to Queue__jki_lib_state_machine.vi"("State(s) in (\"\")"=w293) -> ("States Out"=w292:string)  [unwired: 14 in]
        n169 = Quit LabVIEW() -> ()  [unwired: 1 in]
      }
      frame "--------- Library --------" {
        n170 = call <vilib>:"Add State(s) to Queue__jki_lib_state_machine.vi"("State(s) in (\"\")"=w299) -> ("States Out"=w298:string)  [unwired: 14 in]
      }
      frame "S7: Initialize" {
        n171 = property on="PLC" class="Bool (严格)"("Val(Sgnl)"=FALSE ("值(信号)")) -> ()  [unwired: 2 in, 2 out]
      }
      frame "S7: Stop" {
        n172 = call "Stop Module.vi"("error in (no error)"=w308) -> ("error out"=w307:errorcluster)  [unwired: 10 in]
        n173 = call <vilib>:"Add State(s) to Queue__jki_lib_state_machine.vi"("State(s) in (\"\")"=w309) -> ("States Out"=w310:string)  [unwired: 14 in]
      }
      frame "---------- Data ----------" {
        n174 = call <vilib>:"Add State(s) to Queue__jki_lib_state_machine.vi"("State(s) in (\"\")"=w318) -> ("States Out"=w317:string)  [unwired: 14 in]
      }
      frame "Data: Initialize" {
        w323 = T8 {"Current VI Reference"=refnum, "Close Panel on Exit?"=FALSE}  # Core
        w325 = TRUE  # Your Boolean data
        w324 = ""  # Your string data
        n175 = global write "Global.vi" "程序关闭"(FALSE ("程序关闭")) -> ()
        n176 = global write "Global.vi" "计时开始"(FALSE ("计时结束")) -> ()
        n177 = Bundle("Core"=w323, "Your Boolean data"=w325, "Your string data"=w324) -> (w327:T7)  [unwired: 1 in]
        n178 = call <vilib>:"Add State(s) to Queue__jki_lib_state_machine.vi"("State(s) in (\"\")"=w329) -> ("States Out"=w328:string)  [unwired: 14 in]
      }
      frame "Data: Cleanup" {
        n179 = Unbundle By Name(w332) -> ("Core.Current VI Reference"=w335:refnum<vi>)
        n180 = Close Reference(reference=w335, error in (no error)=w334) -> (error out=w333:errorcluster)
        n181 = call <vilib>:"Add State(s) to Queue__jki_lib_state_machine.vi"("State(s) in (\"\")"=w337) -> ("States Out"=w336:string)  [unwired: 14 in]
      }
      frame "---------- UI ----------" {
        # "Do not put any code in this frame.\n(It is a separator no-op. You can make a copy of this frame to create a new UI frame)"
        n182 = call <vilib>:"Add State(s) to Queue__jki_lib_state_machine.vi"("State(s) in (\"\")"=w343) -> ("States Out"=w342:string)  [unwired: 14 in]
      }
      frame "UI: Initialize" {
        n183 = vi-ref "Auto.vi"() -> (w349:refnum<vi>)
        n184 = invoke class="VI" method="Ctrl Val.Set"(reference=w349, "Control Name"="STEP" ("控件名"), "Value"="初始化" ("控件名")) -> (reference out=w346:refnum<vi>)  [unwired: 2 in, 4 out]
        n185 = disable-structure shown="启用" {
          disable-tunnel: [w363 _] -> w353
          disable-tunnel: w350 -> [w361 _]
          frame Enabled {
            n186 = vi-ref "Auto.vi"() -> (w362:refnum<vi>)
            n187 = property class="VI"(reference=w362) -> (reference out=w360:refnum<vi>, "FP.State"=w359:T2)  [unwired: 1 in, 1 out]
            n188 = case shown="\"Standard\", 默认" w359 {
              tunnel: w361 -> [w369 w371]
              tunnel: w360 -> [w370 w372]
              tunnel: [w368 w372] -> w357
              tunnel: [w367 w371] -> w358
              frame "Standard", Default {
                n189 = invoke class="VI" method="FP.Close"(reference=w370, error in=w369) -> (reference out=w368:refnum<vi>, error out=w367:errorcluster)  [unwired: 1 in, 1 out]
              }
              frame "Invalid", "Closed" {
              }
            }
            n190 = invoke on="子面板" class="SubPnl" method="Insert VI"(error in=w358, "VI Ref"=w357) -> (error out=w366:errorcluster)  [unwired: 2 in, 3 out]
            n191 = invoke class="VI" method="Run VI"(reference=w357, error in=w366, "Wait until done"=FALSE ("结束前等待"), "Auto Dispose Ref"=TRUE ("自动销毁引用")) -> (error out=w363:errorcluster)  [unwired: 1 in, 4 out]
          }
          frame Disabled {
            n192 = vi-ref "Auto.vi"() -> (w374:refnum<vi>)
            n193 = call "CallVI.vi"("VI引用"=w374, "状态"=T2."Maximized") -> ()  [unwired: 11 in, 3 out]
          }
        }
        n194 = invoke class="VI" method="Ctrl Val.Set"(reference=w346, "Control Name"="STEP2" ("控件名"), "Value"="初始化" ("控件名")) -> ()  [unwired: 2 in, 5 out]
        n195 = call <vilib>:"Add State(s) to Queue__jki_lib_state_machine.vi"("State(s) in (\"\")"=w356) -> ("States Out"=w355:string)  [unwired: 14 in]
      }
      frame "UI: Init" {
        n196 = stacked-sequence {
          tunnel: w376 -> [_ _ _ _]
          frame #0 {
            n197 = global write "Global.vi" "程序关闭"(FALSE ("程序关闭")) -> ()
            n198 = vi-ref "状态读取.vi"() -> (w385:refnum<vi>)
            n199 = vi-ref "扭矩.vi"() -> (w384:refnum<vi>)
            n200 = call "CallVI.vi"("VI引用"=w385, "状态"=T2."Hidden") -> ("错误输出"=w383:errorcluster)  [unwired: 11 in, 2 out]
            n201 = call "CallVI.vi"("VI引用"=w384, "状态"=T2."Hidden", "错误输入"=w383) -> ()  [unwired: 10 in, 3 out]
          }
          frame #1 {
            w393 = 0
            n202 = shared-variable "我的电脑\\Global.lvlib\\总成追溯码"("   " ("工位追溯码")) -> ()  [unwired: 1 in, 1 out]
            n203 = global write "Global.vi" "生产数量"(w393) -> ()
            n204 = global write "Global.vi" "合格数量"(w393) -> ()
            n205 = global read "Global1.vi" "用户信息"() -> (w388:T6)
            n206 = global read "Global1.vi" "联机模式"() -> (w387:enum16{"单机", "追溯"})
            n207 = Unbundle By Name(w388) -> ("用户名"=→"userName":string, "用户权限"=→"userStatus":string)
            n208 = case shown="\"追溯\"" w387 {
              tunnel: ["联网" ("connectionMode") "单机" ("connectionMode")] -> w394
              frame "追溯" {
              }
              frame "单机", Default {
              }
            }
            "connectionMode" <- w394
            "产品型号" <- "" ("产品型号")
          }
          frame #2 {
            n209 = control-ref of="表格控件"() -> (w398:refnum<vi>)
            n210 = control-ref of="提示信息"() -> (w400:refnum<vi>)
            n211 = control-ref of="自动"() -> (w401:refnum<vi>)
            n212 = control-ref of="错误"() -> (w402:refnum<vi>)
            n213 = control-ref of="更换产品"() -> (w399:refnum<vi>)
            n214 = global write "Global.vi" "提示信息"(w400) -> ()
            n215 = global write "Global.vi" "程序自动"(w401) -> ()
            n216 = global write "Global.vi" "报警图标"(w402) -> ()
            n217 = global write "Global.vi" "Result"(w398) -> ()
            n218 = global write "Global.vi" "更换产品"(w399) -> ()
            n219 = control-ref of="上序状态"() -> (w397:refnum<vi>)
            n220 = global write "Global.vi" "上序状态"(w397) -> ()
          }
          frame #3 {
            w403 = -2
            n221 = global read "Global.vi" "Result"() -> (w406:refnum<vi>)
            n222 = property class="Tbl"(reference=w406, "Row Headers[]"=string[] [], "Value"=string[][] []) -> ()  [unwired: 1 in, 2 out]
            n223 = Bundle(w403, w403) -> (w404:cluster{i32, i32})  [unwired: 1 in]
            n224 = call "Start_Client.vi"() -> ()  [unwired: 12 in]
            n225 = property class="Tbl"(reference=w406, "Active Cell"=w404, "Cell BG Color"=u32 16777216 ("活动单元格:单元格背景色")) -> ()  [unwired: 1 in, 2 out]
          }
        }
        n226 = call <vilib>:"Add State(s) to Queue__jki_lib_state_machine.vi"("State(s) in (\"\")"=w380) -> ("States Out"=w379:string)  [unwired: 14 in]
      }
      frame "UI: Config" {
        n227 = vi-ref "Config.vi"() -> (w411:refnum<vi>)
        n228 = call "CallVI.vi"("VI引用"=w411, "状态"=T2."Standard") -> ()  [unwired: 11 in, 3 out]
        n229 = call <vilib>:"Add State(s) to Queue__jki_lib_state_machine.vi"("State(s) in (\"\")"=w416) -> ("States Out"=w415:string)  [unwired: 14 in]
      }
      frame "UI: Cursor Set" {
        # "Argument"
        n230 = case shown="\"Idle\", 默认" w419 {
          tunnel: w421 -> [w426 w428]
          tunnel: [w425 w427] -> w420
          frame "Idle", Default {
            n231 = call <vilib>:"Unset Busy.vi"("error in (no error)"=w426) -> ("error out"=w425:errorcluster)  [unwired: 10 in]
          }
          frame "Busy" {
            n232 = call <vilib>:"Set Busy.vi"("error in (no error)"=w428) -> ("error out"=w427:errorcluster)  [unwired: 9 in, 1 out]
          }
        }
        n233 = call <vilib>:"Add State(s) to Queue__jki_lib_state_machine.vi"("State(s) in (\"\")"=w424) -> ("States Out"=w423:string)  [unwired: 14 in]
      }
      frame "UI: Front Panel State" {
        # "Argument"
        n234 = Unbundle By Name(w433) -> ("Core.Current VI Reference"=w432:refnum<vi>)
        n235 = case shown="\"Close\"" w431 {
          tunnel: w435 -> [w441 w454]
          tunnel: [w443 w455] -> w434
          tunnel: w432 -> [w442 w452]
          frame "Open", Default {
            n236 = property class="VI"(reference=w442, error in=w441) -> (reference out=w439:refnum<vi>, error out=w440:errorcluster, "Front Panel.Open"=w438:bool)
            n237 = case shown="假" w438 {
              tunnel: [w446 w449] -> w443
              tunnel: w440 -> [w445 w449]
              tunnel: w439 -> [w444 _]
              frame False {
                n238 = invoke class="VI" method="FP.Open"(reference=w444, error in=w445, "Activate"=TRUE, "State"=T2."Standard") -> (error out=w446:errorcluster)  [unwired: 1 in, 4 out]
              }
              frame True {
              }
            }
          }
          frame "Close" {
            n239 = property class="VI"(reference=w452, error in=w454) -> (reference out=w451:refnum<vi>, error out=w453:errorcluster, "Front Panel.Open"=w450:bool)
            n240 = case shown="真" w450 {
              tunnel: [w456 w459] -> w455
              tunnel: w453 -> [w456 w458]
              tunnel: w451 -> [_ w457]
              frame False {
              }
              frame True {
                n241 = invoke class="VI" method="FP.Close"(reference=w457, error in=w458) -> (error out=w459:errorcluster)  [unwired: 1 in, 2 out]
              }
            }
          }
        }
        n242 = call <vilib>:"Add State(s) to Queue__jki_lib_state_machine.vi"("State(s) in (\"\")"=w437) -> ("States Out"=w436:string)  [unwired: 14 in]
      }
      frame "---------- Macro ----------" {
        n243 = call <vilib>:"Add State(s) to Queue__jki_lib_state_machine.vi"("State(s) in (\"\")"=w465) -> ("States Out"=w464:string)  [unwired: 14 in]
      }
      frame "Macro: Initialize" {
        n244 = call <vilib>:"Add State(s) to Queue__jki_lib_state_machine.vi"("State(s) in Front (\"\")"="Data: Initialize\nInitialize Core Data\nS7: Initialize\nIdle\nUI: Init\nUI: Front Panel State >> Open\nUI: Initialize\nUI: Config", "State(s) in (\"\")"=w472) -> ("States Out"=w471:string)  [unwired: 13 in]
      }
      frame "Macro: Exit" {
        n245 = Unbundle By Name(w481) -> ("Core.Close Panel on Exit?"=w480:bool)
        n246 = Select(t="UI: Front Panel State >> Close", s=w480, f="") -> (s? t:f=w477:string)
        n247 = call <vilib>:"Add State(s) to Queue__jki_lib_state_machine.vi"("State(s) in (\"\")"=w477, "State(s) at Back (\"\")"="Data: Cleanup\nExit") -> ("States Out"=w475:string)  [unwired: 13 in]
        n248 = call <vilib>:"Add State(s) to Queue__jki_lib_state_machine.vi"("State(s) in Front (\"\")"=w475, "State(s) in (\"\")"=w484) -> ("States Out"=w483:string)  [unwired: 13 in]
      }
    }
  }
  n249 = call-dynamic "Cleanup.vi"("MenuStrip in"=w6) -> ()  [unwired: 10 in, 1 out]
